vi "HFRR ADV v039.vi"() -> ()   [LabVIEW 2025] (continued)
            n2168 = Bundle "Bundle"(w2334, w2365) -> (w2352:cluster{dbl[], dbl[]})  [unwired: 1 in]
            n2169 = Bundle "Bundle"(w2334, w2419) -> (w2353:cluster{dbl[], dbl[]})  [unwired: 1 in]
            n2170 = Bundle "Bundle"(w2365, w2361) -> (w2367:cluster{dbl[], dbl[]})  [unwired: 1 in]
            n2171 = Bundle "Bundle"(w2330, w2329) -> (w2337:cluster{dbl[], dbl[]})  [unwired: 1 in]
            n2172 = Bundle "Bundle"(w2363, w2359) -> (w2369:cluster{dbl[], dbl[]})  [unwired: 1 in]
            n2173 = Bundle "Bundle"(w2330, w2363) -> (w2473:cluster{dbl[], dbl[]})  [unwired: 1 in]
            n2174 = Bundle "Bundle"(w2330, w2359) -> (w2397:cluster{dbl[], dbl[]})  [unwired: 1 in]
            n2175 = Bundle "Bundle"(w2330, w2418) -> (w2483:cluster{dbl[], dbl[]})  [unwired: 1 in]
            n2176 = Bundle "Bundle"(w2330, w2413) -> (w2421:cluster{dbl[], dbl[]})  [unwired: 1 in]
            n2177 = Bundle "Bundle"(w2330, w2444) -> (w2468:cluster{dbl[], dbl[]})  [unwired: 1 in]
            n2178 = Bundle "Bundle"(w2364, w2360) -> (w2368:cluster{dbl[], dbl[]})  [unwired: 1 in]
            n2179 = Bundle "Bundle"(w2332, w2331) -> (w2338:cluster{dbl[], dbl[]})  [unwired: 1 in]
            n2180 = Bundle "Bundle"(w2332, w2364) -> (w2475:cluster{dbl[], dbl[]})  [unwired: 1 in]
            n2181 = Bundle "Bundle"(w2332, w2360) -> (w2398:cluster{dbl[], dbl[]})  [unwired: 1 in]
            n2182 = Bundle "Bundle"(w2332, w2414) -> (w2422:cluster{dbl[], dbl[]})  [unwired: 1 in]
            n2183 = Bundle "Bundle"(w2332, w2416) -> (w2484:cluster{dbl[], dbl[]})  [unwired: 1 in]
            n2184 = Bundle "Bundle"(w2332, w2453) -> (w2466:cluster{dbl[], dbl[]})  [unwired: 1 in]
            n2185 = Bundle "Bundle"(w2362, w2358) -> (w2370:cluster{dbl[], dbl[]})  [unwired: 1 in]
            n2186 = Bundle "Bundle"(w2328, w2327) -> (w2336:cluster{dbl[], dbl[]})  [unwired: 1 in]
            n2187 = Bundle "Bundle"(w2328, w2362) -> (w2474:cluster{dbl[], dbl[]})  [unwired: 1 in]
            n2188 = Bundle "Bundle"(w2328, w2358) -> (w2396:cluster{dbl[], dbl[]})  [unwired: 1 in]
            n2189 = Bundle "Bundle"(w2328, w2412) -> (w2420:cluster{dbl[], dbl[]})  [unwired: 1 in]
            n2190 = Bundle "Bundle"(w2328, w2417) -> (w2482:cluster{dbl[], dbl[]})  [unwired: 1 in]
            n2191 = Bundle "Bundle"(w2328, w2435) -> (w2467:cluster{dbl[], dbl[]})  [unwired: 1 in]
            n2192 = call-poly <vilib>:"Mean.vi"("X"=w2415) -> ("mean"=→"CP1":dbl)  [unwired: 1 out]
            n2193 = call-poly <vilib>:"Mean.vi"("X"=w2356) -> ("mean"=→"КОФ2 3":dbl)  [unwired: 1 out]
            n2194 = call-poly <vilib>:"Mean.vi"("X"=w2414) -> ("mean"=→"CP2":dbl)  [unwired: 1 out]
            n2195 = call-poly <vilib>:"Mean.vi"("X"=w2416) -> ("mean"=→"КОФ2":dbl)  [unwired: 1 out]
            n2196 = call-poly <vilib>:"Mean.vi"("X"=w2354) -> ("mean"=→"КОФ2 5":dbl)  [unwired: 1 out]
            n2197 = call-poly <vilib>:"Mean.vi"("X"=w2412) -> ("mean"=→"CP4":dbl)  [unwired: 1 out]
            n2198 = call-poly <vilib>:"Mean.vi"("X"=w2417) -> ("mean"=→"КОФ4":dbl)  [unwired: 1 out]
            n2199 = Bundle "Bundle"(w2334, w2361) -> (w2325:cluster{dbl[], dbl[]})  [unwired: 1 in]
            n2200 = Bundle "Bundle"(w2334, w2415) -> (w2348:cluster{dbl[], dbl[]})  [unwired: 1 in]
            n2201 = Build Array "Build Array"(w2325, w2348) -> (w2351:cluster{dbl[], dbl[]}[])
            "XY Graph 17" <- w2351
            n2202 = Build Array "Build Array"(w2339, w2338, w2337, w2336) -> (→"Frequency ( Hz )":cluster{dbl[], dbl[]}[])
            n2203 = Build Array "Build Array"(w2367, w2368, w2369, w2370) -> (→"Air Temp ( °C ) vs Humidity ( % RH )":cluster{dbl[], dbl[]}[])
            n2204 = Build Array "Build Array"(w2352, w2475, w2473, w2474) -> (→"Air Temperature  ( °C )":cluster{dbl[], dbl[]}[])
            n2205 = Build Array "Build Array"(w2325, w2398, w2397, w2396) -> (→"Humidity ( %RH )":cluster{dbl[], dbl[]}[])
            n2206 = Build Array "Build Array"(w2353, w2484, w2483, w2482) -> (→"Coefficient Of Friction":cluster{dbl[], dbl[]}[])
            n2207 = Build Array "Build Array"(w2348, w2422, w2421, w2420) -> (→"Sample Temperature ( °C )":cluster{dbl[], dbl[]}[])
            n2208 = Build Array "Build Array"(w2326, w2466, w2468, w2467) -> (→"XY Graph 13":cluster{dbl[], dbl[]}[])
            n2209 = Bundle "Bundle"(w2334, w2357) -> (w2379:cluster{dbl[], dbl[]})  [unwired: 1 in]
            n2210 = Bundle "Bundle"(w2330, w2355) -> (w2377:cluster{dbl[], dbl[]})  [unwired: 1 in]
            n2211 = Bundle "Bundle"(w2332, w2356) -> (w2378:cluster{dbl[], dbl[]})  [unwired: 1 in]
            n2212 = Bundle "Bundle"(w2328, w2354) -> (w2376:cluster{dbl[], dbl[]})  [unwired: 1 in]
            n2213 = Build Array "Build Array"(w2379, w2378, w2377, w2376) -> (→"Stroke ( mm )":cluster{dbl[], dbl[]}[])
            n2214 = local write "XY Graph 16"(w2351) -> ()
          }
          frame #2 {
          }
          frame #3 {
            n2215 = local write "Numeric 8"(0 ("Numeric 8")) -> ()
            n2216 = local write "Numeric 11"(0 ("Numeric 11")) -> ()
            n2217 = local write "Numeric 12"(0 ("Numeric 12")) -> ()
            n2218 = local write "Numeric 13"(0 ("Numeric 13")) -> ()
            n2219 = property on="OPEN" class="Bool (strict)"("Visible"=TRUE) -> ()  [unwired: 2 in, 2 out]
            n2220 = local read "String Control 2"() -> (w2651:string)
            n2221 = local read "String Control 4"() -> (w2650:string)
            n2222 = local read "String Control 6"() -> (w2649:string)
            n2223 = local read "String Control 8"() -> (w2648:string)
            n2224 = Match Pattern(string=w2651, regular expression="Samples / cycle :- ") -> (after substring=w2665:string)  [unwired: 1 in, 3 out]
            n2225 = Match Pattern(string=w2651, regular expression="Frequency :- ") -> (after substring=w2684:string)  [unwired: 1 in, 3 out]
            n2226 = Match Pattern(string=w2650, regular expression="Samples / cycle :- ") -> (after substring=w2661:string)  [unwired: 1 in, 3 out]
            n2227 = Match Pattern(string=w2650, regular expression="Frequency :- ") -> (after substring=w2679:string)  [unwired: 1 in, 3 out]
            n2228 = Match Pattern(string=w2649, regular expression="Samples / cycle :- ") -> (after substring=w2657:string)  [unwired: 1 in, 3 out]
            n2229 = Match Pattern(string=w2649, regular expression="Frequency :- ") -> (after substring=w2674:string)  [unwired: 1 in, 3 out]
            n2230 = Match Pattern(string=w2648, regular expression="Samples / cycle :- ") -> (after substring=w2653:string)  [unwired: 1 in, 3 out]
            n2231 = Match Pattern(string=w2648, regular expression="Frequency :- ") -> (after substring=w2669:string)  [unwired: 1 in, 3 out]
            n2232 = String Subset(string=w2665, length (rest)=6 ("length (rest)")) -> (substring=w2667:string)  [unwired: 1 in]
            n2233 = String Subset(string=w2684, length (rest)=9 ("length (rest)")) -> (substring=w2686:string)  [unwired: 1 in]
            n2234 = String Subset(string=w2661, length (rest)=6 ("length (rest)")) -> (substring=w2663:string)  [unwired: 1 in]
            n2235 = String Subset(string=w2679, length (rest)=9 ("length (rest)")) -> (substring=w2681:string)  [unwired: 1 in]
            n2236 = String Subset(string=w2657, length (rest)=6 ("length (rest)")) -> (substring=w2659:string)  [unwired: 1 in]
            n2237 = String Subset(string=w2674, length (rest)=9 ("length (rest)")) -> (substring=w2676:string)  [unwired: 1 in]
            n2238 = String Subset(string=w2653, length (rest)=6 ("length (rest)")) -> (substring=w2655:string)  [unwired: 1 in]
            n2239 = String Subset(string=w2669, length (rest)=9 ("length (rest)")) -> (substring=w2671:string)  [unwired: 1 in]
            n2240 = Fract/Exp String To Number(string=w2667) -> (number=w2647:dbl)  [unwired: 3 in, 1 out]
            n2241 = Fract/Exp String To Number(string=w2686) -> (number=w2687:dbl)  [unwired: 3 in, 1 out]
            n2242 = Fract/Exp String To Number(string=w2663) -> (number=w2646:dbl)  [unwired: 3 in, 1 out]
            n2243 = Fract/Exp String To Number(string=w2681) -> (number=w2682:dbl)  [unwired: 3 in, 1 out]
            n2244 = Fract/Exp String To Number(string=w2659) -> (number=w2645:dbl)  [unwired: 3 in, 1 out]
            n2245 = Fract/Exp String To Number(string=w2676) -> (number=w2677:dbl)  [unwired: 3 in, 1 out]
            n2246 = Fract/Exp String To Number(string=w2655) -> (number=w2644:dbl)  [unwired: 3 in, 1 out]
            n2247 = Fract/Exp String To Number(string=w2671) -> (number=w2672:dbl)  [unwired: 3 in, 1 out]
            n2248 = local write "sample1"(w2647) -> ()
            n2249 = local write "freq1"(w2687) -> ()
            n2250 = local write "sample2"(w2646) -> ()
            n2251 = local write "freq2"(w2682) -> ()
            n2252 = local write "sample3"(w2645) -> ()
            n2253 = local write "freq3"(w2677) -> ()
            n2254 = local write "sample4"(w2644) -> ()
            n2255 = local write "freq 4"(w2672) -> ()
          }
        }
      }
    }
    n2256 = case shown="True" w2245 {
      selector: w2245 -> [_ w2264]
      frame False {
      }
      frame True {
        n2257 = Not(x=w2264) -> (.not. x?=w2260:bool)
        n2258 = local write "service 3"(w2260) -> ()
        n2259 = local write "OPEN 6"(w2260) -> ()
        n2260 = call <vilib>:"System Exec.vi"("wait until completion? (T)"=TRUE, "command line"="C:\\LAB-IQ\\Scar View.exe") -> ("error out"=→"error out 5":errorcluster)  [unwired: 6 in, 3 out]
      }
    }
    n2261 = case shown="\"Acquire\", Default" w2254 {
      frame "Acquire", Default {
        # "Elapsed time\ncof\nstroke\nAir temp\nTemp\nHumidity"
        n2262 = disable-structure shown="Disabled" {
          frame Disabled {
            n2263 = local read "Flag"() -> (w2963:dbl)
            n2264 = local read "RUN"() -> (w2960:bool)
            n2265 = Not(x=w2960) -> (.not. x?=w2959:bool)
            n2266 = Equal?(x=w2963, y=10.0) -> (x = y?=w2961:bool)
            n2267 = And(x=w2961, y=w2959) -> (x .and. y?=w2958:bool)
            n2268 = case shown="True" w2958 {
              frame False {
              }
              frame True {
                w2964 = FALSE ("Heater Button")
                n2269 = local write "Humidity"(w2964) -> ()
                n2270 = local write "Heater Button"(w2964) -> ()
              }
            }
          }
          frame Enabled {
          }
        }
        n2271 = disable-structure shown="Disabled" {
          frame Disabled {
            n2272 = case shown="True" {
              selector: _ -> [_ _]
              frame False {
              }
              frame True {
                w3009 = TRUE ("Heater")
                n2273 = local write "Humidity"(w3009) -> ()
                n2274 = local write "Heater Button"(w3009) -> ()
                n2275 = local read "TEST STANDARD"() -> (w3012:T3)
                n2276 = local read "TEST STANDARD"() -> (w3007:T3)
                n2277 = Equal?(x=w3012, y=enum16{"ASTM D6079", "ISO 12156", "Custom"}."ISO 12156" ("Test Standard")) -> (x = y?=w3010:bool)
                n2278 = Equal?(x=w3007, y=enum16{"ASTM D6079", "ISO 12156", "Custom"}."ASTM D6079" ("Test Standard")) -> (x = y?=w3006:bool)
                n2279 = case shown="True" w3010 {
                  frame False {
                  }
                  frame True {
                    n2280 = local write "airtempflg"(FALSE ("airtempflg")) -> ()
                    n2281 = local write item#-1(TRUE ("Heater")) -> ()
                  }
                }
                n2282 = case shown="True" w3006 {
                  frame False {
                  }
                  frame True {
                    n2283 = local write "airtempflg"(TRUE ("airtempflg")) -> ()
                    n2284 = local write item#-1(FALSE ("Heater")) -> ()
                  }
                }
              }
            }
          }
          frame Enabled {
          }
        }
        n2285 = stacked-sequence {
          frame #0 {
            n2286 = case shown="True" "RST FF" {
              frame False {
              }
              frame True {
                w3026 = 0.0 ("X Scale.Range:Maximum")
                n2287 = property on="Frictional Force ( N )" class="WFChart (strict)"("XScale.Maximum"=600.0 ("X Scale.Range:Maximum"), "XScale.Minimum"=w3026, "YScale.Maximum"=10.0 ("Y Scale.Range:Maximum"), "YScale.Minimum"=w3026) -> ()  [unwired: 2 in, 2 out]
              }
            }
          }
          frame #1 {
            n2288 = case shown="True" "RST TEMP" {
              frame False {
              }
              frame True {
                n2289 = property on="Temperature ( Deg C )" class="WFChart (strict)"("XScale.Minimum"=0.0 ("X Scale.Range:Minimum"), "XScale.Maximum"=600.0 ("X Scale.Range:Maximum"), "YScale.Minimum"=0.0 ("Y Scale.Range:Minimum"), "YScale.Maximum"=100.0 ("Y Scale.Range:Maximum")) -> ()  [unwired: 2 in, 2 out]
              }
            }
          }
          frame #2 {
            n2290 = case shown="True" "RSTCOF" {
              frame False {
              }
              frame True {
                n2291 = property on="Coefficient of Friction" class="WFChart (strict)"("XScale.Minimum"=0.0 ("X Scale.Range:Minimum"), "XScale.Maximum"=600.0 ("X Scale.Range:Maximum"), "YScale.Maximum"=1.0 ("X Scale.Range:Minimum"), "YScale.Minimum"=0.0 ("X Scale.Range:Minimum")) -> ()  [unwired: 2 in, 2 out]
              }
            }
          }
          frame #3 {
            n2292 = case shown="True" "RSTCOF 2" {
              frame False {
              }
              frame True {
                (unwired) 100.0 ("Y Scale.Range:Maximum")
                (unwired) 0.0 ("Y Scale.Range:Minimum")
                (unwired) 600.0 ("X Scale.Range:Maximum")
                (unwired) 0.0 ("X Scale.Range:Minimum")
              }
            }
          }
          frame #4 {
            n2293 = case shown="True" "RSTCOF 3" {
              frame False {
              }
              frame True {
                n2294 = property on="Electrical Contact Resistance ( % )" class="WFChart (strict)"("XScale.Minimum"=0.0 ("X Scale.Range:Minimum"), "XScale.Maximum"=600.0 ("X Scale.Range:Maximum"), "YScale.Minimum"=0.0 ("Y Scale.Range:Minimum"), "YScale.Maximum"=100.0 ("Y Scale.Range:Maximum")) -> ()  [unwired: 2 in, 2 out]
              }
            }
          }
        }
        n2295 = local read "RUN"() -> (w2953:bool)
        n2296 = case shown="False" w2953 {
          frame False {
          }
          frame True {
          }
        }
        n2297 = local read "RUN"() -> (w2957:bool)
        n2298 = case shown="False" w2957 {
          tunnel: [FALSE ("TEST RUNNING") TRUE ("TEST RUNNING")] -> w2956
          frame False {
            w3045 = 0.0 ("Flag")
            n2299 = local write "Elapsed time"(0.0 ("elapsedtime")) -> ()
            n2300 = local write "Time Remaining"(w3045) -> ()
            n2301 = local write "Flag"(w3045) -> ()
            n2302 = local write "Remaining Time"(w3045) -> ()
          }
          frame True {
            n2303 = local write "Flag"(10.0 ("Flag")) -> ()
          }
        }
        n2304 = local read "AIR TEMP"() -> (w2951:dbl)
        n2305 = Greater Or Equal?(x=w2951, y=15.0) -> (x >= y?=w2952:bool)
        "powstat" <- w2952
        n2306 = case shown="True" "Save & Continue" {
          frame False {
          }
          frame True {
            n2307 = local read "USER ID"() -> (w3349:string)
            n2308 = local read "FILE"() -> (w3357:string)
            n2309 = String Length(string=w3357) -> (length=w3355:i32)
            n2310 = String Length(string=w3349) -> (length=w3352:i32)
            n2311 = Greater?(x=w3355, y=0) -> (0:w3354:bool)
            n2312 = Greater?(x=w3352, y=0) -> (0:w3351:bool)
            n2313 = And(x=w3354, y=w3351) -> (x .and. y?=w3350:bool)
            n2314 = case shown="True" w3350 {
              frame False {
                n2315 = stacked-sequence {
                  frame #0 {
                    n2316 = One Button Dialog(message="Please Enter a File Name and Operator ID to save data !", button name ("OK")="Ok") -> ()  [unwired: 1 out]
                  }
                  frame #1 {
                    n2317 = local write "Save & Continue"(FALSE ("OK Button")) -> ()
                  }
                }
                n2318 = local write "Save & Continue"(FALSE ("OK Button")) -> ()
              }
              frame True {
                n2319 = stacked-sequence {
                  frame #0 {
                    n2320 = local read "FILE"() -> (w3363:string)
                    n2321 = call "file check.vi"("file name in"=w3363) -> ("file name out"=w3362:string)  [unwired: 9 in, 1 out]
                    n2322 = call <vilib>:"Application Directory.vi"() -> ("Application Directory"=w3373:path)
                    n2323 = Build Path(base path=w3373, name or relative path="data") -> (appended path=w3372:path)
                    n2324 = call <vilib>:"Trim Whitespace.vi"("string"=w3362) -> ("trimmed string"=w3370:string)  [unwired: 1 in]
                    n2325 = call <vilib>:"Trim Whitespace.vi"("string"=w3362) -> ("trimmed string"=w3371:string)  [unwired: 1 in]
                    n2326 = List Folder(path=w3372) -> (folder names=w3368:string[])  [unwired: 3 in, 3 out]
                    n2327 = Match Pattern(string=w3370, regular expression="_(") -> (before substring=w3367:string)  [unwired: 1 in, 3 out]
                    n2328 = for {
                      tunnel: w3368 -> [w3382] mode=indexing
                      tunnel: w3367 -> [w3380]
                      shift-right: [w3378] -> w3365
                      shift-left: bool[] [] -> [w3379]
                      n2329 = Match Pattern(string=w3382, regular expression="_(") -> (before substring=w3381:string)  [unwired: 1 in, 3 out]
                      n2330 = Equal?(x=w3381, y=w3380) -> (x = y?=w3377:bool)
                      n2331 = case shown="True" w3377 {
                        tunnel: w3377 -> [_ w3385]
                        tunnel: w3379 -> [w3384 w3387]
                        tunnel: [w3384 w3386] -> w3378
                        frame False {
                        }
                        frame True {
                          n2332 = Insert Into Array(array=w3387, new element=w3385) -> (w3386:bool[])  [unwired: 1 in]
                        }
                      }
                    }
                    n2333 = Equal?(x=w3368, y=w3367) -> (x = y?=w3376:bool[])
                    n2334 = Or Array Elements(Boolean array=w3376) -> (logical OR=w3375:bool)
                    n2335 = Array Size(array=w3365) -> (size(s)=w3364:i32)
                    n2336 = case shown="True" w3375 {
                      tunnel: w3371 -> [_ w3395]
                      tunnel: w3364 -> [_ w3388]
                      frame False {
                      }
                      frame True {
                        n2337 = Number To Decimal String(number=w3388) -> (decimal integer string=w3391:string)  [unwired: 1 in]
                        n2338 = Search/Split String(string=w3395, search string/char (-)="_(" ("regular expression")) -> (substring before match=w3393:string)  [unwired: 1 in, 2 out]
                        n2339 = Concatenate Strings(w3393, "_(" ("regular expression"), w3391, ")" ("regular expression")) -> (w3389:string)
                        n2340 = local write "FILE"(w3389) -> ()
                      }
                    }
                  }
                  frame #1 {
                    w3398 = 0.0
                    w3411 = cluster{"y":dbl, dbl, "y":dbl}[] [] ("History Data")
                    w3412 = FALSE ("Heater Button")
                    (unwired) ")!" ("string")
                    (unwired) ")" ("string")
                    w3410 = dbl[] [] ("History Data")
                    w3416 = "\r"
                    # "C:\\WinDucom\\Data\\"
                    # "C:\\LAB-IQ-NXT\\data"
                    n2341 = local write "Humidity ( %RH )"(w3398) -> ()
                    n2342 = local write "Frequency ( Hz )"(w3398) -> ()
                    n2343 = local write "Stroke 3"(w3398) -> ()
                    n2344 = local write "speedop"(0.0 ("PIDclk 2")) -> ()
                    n2345 = local write "Set Temp 2"(65.0 ("Set Temp 2")) -> ()
                    n2346 = local write "AIR TEMP"(w3398) -> ()
                    n2347 = local write "clk"(0.0 ("clk")) -> ()
                    n2348 = local write "Stroke 4"(w3398) -> ()
                    n2349 = local write "COF 2"(w3398) -> ()
                    n2350 = local write "TEMP"(w3398) -> ()
                    n2351 = local write "ecr 3"(w3398) -> ()
                    n2352 = local write "FF 3"(w3398) -> ()
                    n2353 = local write "FF 2"(w3398) -> ()
                    n2354 = property on="Coefficient of Friction" class="WFChart (strict)"("History Data"=w3410) -> ()  [unwired: 2 in, 2 out]
                    n2355 = property on="Coefficient of Friction" class="WFChart (strict)"("History Data"=w3410) -> ()  [unwired: 2 in, 2 out]
                    n2356 = property on="Frictional Force ( N )" class="WFChart (strict)"("History Data"=w3410) -> ()  [unwired: 2 in, 2 out]
                    n2357 = property on="Electrical Contact Resistance ( % )" class="WFChart (strict)"("History Data"=w3410) -> ()  [unwired: 2 in, 2 out]
                    n2358 = property on="Electrical Contact Resistance ( % )" class="WFChart (strict)"("History Data"=w3410) -> ()  [unwired: 2 in, 2 out]
                    n2359 = property on="Temperature ( Deg C )" class="WFChart (strict)"("History Data"=w3410) -> ()  [unwired: 2 in, 2 out]
                    n2360 = property on="Frictional Force ( N )" class="WFChart (strict)"("History Data"=w3410) -> ()  [unwired: 2 in, 2 out]
                    n2361 = property on="Coefficient of Friction" class="WFChart (strict)"("History Data"=w3410) -> ()  [unwired: 2 in, 2 out]
                    n2362 = property on="Frictional Force ( N )" class="WFChart (strict)"("History Data"=w3410) -> ()  [unwired: 2 in, 2 out]
                    n2363 = property on="Electrical Contact Resistance ( % )" class="WFChart (strict)"("History Data"=w3410) -> ()  [unwired: 2 in, 2 out]
                    n2364 = property on="Temperature ( Deg C )" class="WFChart (strict)"("History Data"=w3410) -> ()  [unwired: 2 in, 2 out]
                    n2365 = property on="Stroke ( mm )" class="WFChart (strict)"("History Data"=w3411) -> ()  [unwired: 2 in, 2 out]
                    n2366 = property on="Stroke ( mm )" class="WFChart (strict)"("History Data"=w3411) -> ()  [unwired: 2 in, 2 out]
                    n2367 = local write "Humidity"(w3412) -> ()
                    n2368 = local write "Heater Button"(w3412) -> ()
                    n2369 = local read "FILE"() -> (w3406:string)
                    n2370 = disable-structure shown="Enabled" {
                      disable-tunnel: [w3450 _] -> w3397
                      frame Enabled {
                        n2371 = local read "NORMAL LOAD"() -> (w3450:dbl)
                      }
                      frame Disabled {
                      }
                    }
                    n2372 = call "file check.vi"("file name in"=w3406) -> ("error out"=w3409:errorcluster, "file name out"=w3403:string)  [unwired: 9 in]
                    n2373 = call "FILE PATH CREATION.vi"("error in"=w3409, "FILE NAME :"=w3403) -> ("FILE OUT"=w3402:path)  [unwired: 8 in, 1 out]
                    n2374 = Concatenate Strings(w3403, ".dgf" ("Substring")) -> (w3408:string)
                    n2375 = Concatenate Strings(w3403, ".duf" ("Substring")) -> (w3404:string)
                    n2376 = Multiply(x=w3397, y=1.0) -> (x*y=w3429:dbl)
                    n2377 = Build Path(base path=w3402, name or relative path=w3408) -> (appended path=w3401:path)
                    n2378 = Build Path(base path=w3402, name or relative path=w3404) -> (appended path=w3400:path)
                    n2379 = Number To Fractional String(number=w3429, width (-)=i16 5, precision (6)=i16 2) -> (F-format string=w3437:string)  [unwired: 1 in]
                    n2380 = local read "tested by"() -> (w3396:string)
                    n2381 = local read "Fuel Discription :"() -> (w3425:string)
                    n2382 = local read "Batch Ref Num :"() -> (w3414:string)
                    n2383 = Get Date/Time String(date format (0)=enum16{"short", "long", "abbreviated"}."short") -> (date string=w3448:string, time string=w3445:string)  [unwired: 2 in]
                    n2384 = local read "Remarks :"() -> (w3424:string)
                    n2385 = Concatenate Strings("Load :- " ("Substring"), w3437, " grams ," ("Substring")) -> (w3436:string)
                    n2386 = local read "String 41"() -> (w3417:string)
                    n2387 = Concatenate Strings(w3425) -> (w3426:string)
                    n2388 = Concatenate Strings(w3414) -> (w3413:string)
                    n2389 = Concatenate Strings(w3396) -> (w3420:string)
                    n2390 = Concatenate Strings("(" ("Substring"), w3448, ")" ("Substring"), w3445) -> (w3419:string)
                    "concatenated string" <- w3419
                    n2391 = Concatenate Strings(w3424, "," ("string")) -> (w3423:string)
                    n2392 = Concatenate Strings("  TIME;      COF;       STROKE;     AIR TEMP;  TEMP;  HUMIDITY;  ECR; PID-OUT; FREQUENCY" ("Substring"), "\r") -> (w3432:string)
                    n2393 = Concatenate Strings(w3417, w3416, "Fuel Discription :-" ("Substring"), w3426, w3416, w3436, w3416, "Batch Ref Num :-" ("Substring"), w3413, w3416, " Remarks :- " ("Substring"), w3423, w3416, " Date :- " ("Substring"), w3419, w3416, "Tested By :-" ("Substring"), w3420) -> (w3430:string)
                    "REMARKS" <- w3430
                    n2394 = call <vilib>:"Write Characters To File.vi"("append to file? (new file:F)"=FALSE, "character string"=w3432, "file path (dialog if empty)"=w3401) -> ()  [unwired: 2 in, 1 out]
                    n2395 = call <vilib>:"Write Characters To File.vi"("append to file? (new file:F)"=FALSE, "character string"=w3430, "file path (dialog if empty)"=w3400) -> ()  [unwired: 2 in, 1 out]
                  }
                  frame #2 {
                    n2396 = local write "Cycles elapsed"(0 ("Cycles elapsed")) -> ()
                    n2397 = local write "cyclecount"(0 ("cyclecount")) -> ()
                    n2398 = local write "Save & Continue"(FALSE ("OK")) -> ()
                    n2399 = local write "autostrtflg"(TRUE ("autostrtflg")) -> ()
                    n2400 = local write "Save"(FALSE ("Save")) -> ()
                    n2401 = Get Date/Time In Seconds() -> (seconds since 1Jan1904=w3455:timestamp)
                    n2402 = To Double Precision Float(number=w3455) -> (double precision float=w3454:dbl)
                    n2403 = local write "acq timer"(w3454) -> ()
                    n2404 = One Button Dialog(message="Please ensure sample is mounted properly and machine is ready in all aspects for testing !", button name ("OK")="Ok") -> ()  [unwired: 1 out]
                  }
                  frame #3 {
                    n2405 = stacked-sequence {
                      frame #0 {
                        n2406 = local write "Main Dashboard Buttons"(T1."Dashboard" ("Main Dashboard Buttons")) -> ()
                        n2407 = local write "Main Tab"(T2."Acquire" ("Main Tab")) -> ()
                      }
                      frame #1 {
                        n2408 = local write "EVENT LOG"("" ("EVENT LOG")) -> ()
                      }
                      frame #2 {
                        n2409 = Wait (ms)(milliseconds to wait=u32 50) -> ()  [unwired: 1 out]
                      }
                      frame #3 {
                        n2410 = disable-structure shown="Disabled" {
                          frame Disabled {
                            n2411 = local read "EVENT LOG"() -> (w3467:string)
                            n2412 = call "Event Log.vi"("Content"="Test Details", "EVENT LOG"=w3467) -> ("EVENT LOG"=w3466:string)  [unwired: 8 in, 1 out]
                            n2413 = local write "EVENT LOG"(w3466) -> ()
                          }
                          frame Enabled {
                          }
                        }
                      }
                      frame #4 {
                        n2414 = Wait (ms)(milliseconds to wait=u32 50) -> ()  [unwired: 1 out]
                      }
                      frame #5 {
                        n2415 = local read "FILE"() -> (w3469:string)
                        n2416 = Concatenate Strings("File Name :" ("Content"), w3469) -> (w3470:string)
                        n2417 = local read "EVENT LOG"() -> (w3473:string)
                        n2418 = call "Event Log.vi"("Content"=w3470, "EVENT LOG"=w3473) -> ("EVENT LOG"=w3472:string)  [unwired: 8 in, 1 out]
                        n2419 = local write "EVENT LOG"(w3472) -> ()
                      }
                      frame #6 {
                        n2420 = Wait (ms)(milliseconds to wait=u32 50) -> ()  [unwired: 1 out]
                      }
                      frame #7 {
                        n2421 = local read "Batch Ref Num :"() -> (w3475:string)
                        n2422 = Concatenate Strings("Batch Ref No :" ("Content"), w3475) -> (w3476:string)
                        n2423 = local read "EVENT LOG"() -> (w3479:string)
                        n2424 = call "Event Log.vi"("Content"=w3476, "EVENT LOG"=w3479) -> ("EVENT LOG"=w3478:string)  [unwired: 8 in, 1 out]
                        n2425 = local write "EVENT LOG"(w3478) -> ()
                      }
                      frame #8 {
                        n2426 = Wait (ms)(milliseconds to wait=u32 50) -> ()  [unwired: 1 out]
                      }
                      frame #9 {
                        n2427 = local read "tested by"() -> (w3481:string)
                        n2428 = Concatenate Strings("Tested By :" ("Content"), w3481) -> (w3482:string)
                        n2429 = local read "EVENT LOG"() -> (w3485:string)
                        n2430 = call "Event Log.vi"("Content"=w3482, "EVENT LOG"=w3485) -> ("EVENT LOG"=w3484:string)  [unwired: 8 in, 1 out]
                        n2431 = local write "EVENT LOG"(w3484) -> ()
                      }
                      frame #10 {
                        n2432 = Wait (ms)(milliseconds to wait=u32 50) -> ()  [unwired: 1 out]
                      }
                      frame #11 {
                        n2433 = local read "TEST STANDARD"() -> (w3488:T3)
                        n2434 = case shown="\"ASTM D6079\", Default" w3488 {
                          tunnel: ["ASTM D6079" "ISO 12156" "CEC F-096-A-06" "Custom"] -> w3487
                          frame "ASTM D6079", Default {
                          }
                          frame "ISO 12156" {
                          }
                          frame "CEC F-096-A-06" {
                          }
                          frame "Custom" {
                          }
                        }
                        n2435 = Concatenate Strings("Test Standard :" ("Content"), w3487) -> (w3489:string)
                        n2436 = local read "EVENT LOG"() -> (w3492:string)
                        n2437 = call "Event Log.vi"("Content"=w3489, "EVENT LOG"=w3492) -> ("EVENT LOG"=w3491:string)  [unwired: 8 in, 1 out]
                        n2438 = local write "EVENT LOG"(w3491) -> ()
                      }
                      frame #12 {
                        n2439 = Wait (ms)(milliseconds to wait=u32 50) -> ()  [unwired: 1 out]
                      }
                      frame #13 {
                        n2440 = local read "Fuel Discription :"() -> (w3498:string)
                        n2441 = Concatenate Strings("Fuel Description :" ("Content"), w3498) -> (w3499:string)
                        n2442 = local read "EVENT LOG"() -> (w3502:string)
                        n2443 = call "Event Log.vi"("Content"=w3499, "EVENT LOG"=w3502) -> ("EVENT LOG"=w3501:string)  [unwired: 8 in, 1 out]
                        n2444 = local write "EVENT LOG"(w3501) -> ()
                      }
                      frame #14 {
                        n2445 = Wait (ms)(milliseconds to wait=u32 50) -> ()  [unwired: 1 out]
                      }
                      frame #15 {
                        n2446 = local read "Remarks :"() -> (w3504:string)
                        n2447 = Concatenate Strings("Remarks :" ("Content"), w3504) -> (w3505:string)
                        n2448 = local read "EVENT LOG"() -> (w3508:string)
                        n2449 = call "Event Log.vi"("Content"=w3505, "EVENT LOG"=w3508) -> ("EVENT LOG"=w3507:string)  [unwired: 8 in, 1 out]
                        n2450 = local write "EVENT LOG"(w3507) -> ()
                      }
                      frame #16 {
                        n2451 = Wait (ms)(milliseconds to wait=u32 50) -> ()  [unwired: 1 out]
                      }
                      frame #17 {
                        n2452 = local read "USER ID"() -> (w3510:string)
                        n2453 = Concatenate Strings("Operator ID :" ("Content"), w3510) -> (w3512:string)
                        n2454 = local read "EVENT LOG"() -> (w3514:string)
                        n2455 = call "Event Log.vi"("Content"=w3512, "EVENT LOG"=w3514) -> ("EVENT LOG"=w3513:string)  [unwired: 8 in, 1 out]
                        n2456 = local write "EVENT LOG"(w3513) -> ()
                      }
                      frame #18 {
                        n2457 = Wait (ms)(milliseconds to wait=u32 50) -> ()  [unwired: 1 out]
                      }
                      frame #19 {
                        n2458 = disable-structure shown="Disabled" {
                          frame Disabled {
                            n2459 = local read "EVENT LOG"() -> (w3518:string)
                            n2460 = call "Event Log.vi"("Content"="Test Parameter", "EVENT LOG"=w3518) -> ("EVENT LOG"=w3517:string)  [unwired: 8 in, 1 out]
                            n2461 = local write "EVENT LOG"(w3517) -> ()
                          }
                          frame Enabled {
                          }
                        }
                      }
                      frame #20 {
                        n2462 = Wait (ms)(milliseconds to wait=u32 50) -> ()  [unwired: 1 out]
                      }
                      frame #21 {
                        n2463 = local read "Set Hz"() -> (w3522:dbl)
                        n2464 = Number To Fractional String(number=w3522, precision (6)=i16 2) -> (F-format string=w3521:string)  [unwired: 2 in]
                        n2465 = Concatenate Strings("Set Frequency [Hz] :" ("Content"), w3521) -> (w3524:string)
                        n2466 = local read "EVENT LOG"() -> (w3526:string)
                        n2467 = call "Event Log.vi"("Content"=w3524, "EVENT LOG"=w3526) -> ("EVENT LOG"=w3525:string)  [unwired: 8 in, 1 out]
                        n2468 = local write "EVENT LOG"(w3525) -> ()
                      }
                      frame #22 {
                        n2469 = Wait (ms)(milliseconds to wait=u32 50) -> ()  [unwired: 1 out]
                      }
                      frame #23 {
                        n2470 = local read "NORMAL LOAD"() -> (w3529:dbl)
                        n2471 = Number To Fractional String(number=w3529, precision (6)=i16 2) -> (F-format string=w3530:string)  [unwired: 2 in]
                        n2472 = Concatenate Strings("Applied Load [grams] :" ("Content"), w3530) -> (w3532:string)
                        n2473 = local read "EVENT LOG"() -> (w3534:string)
                        n2474 = call "Event Log.vi"("Content"=w3532, "EVENT LOG"=w3534) -> ("EVENT LOG"=w3533:string)  [unwired: 8 in, 1 out]
                        n2475 = local write "EVENT LOG"(w3533) -> ()
                      }
                      frame #24 {
                        n2476 = Wait (ms)(milliseconds to wait=u32 50) -> ()  [unwired: 1 out]
                      }
                      frame #25 {
                        n2477 = local read "Set Strk"() -> (w3537:dbl)
                        n2478 = Number To Fractional String(number=w3537, precision (6)=i16 2) -> (F-format string=w3538:string)  [unwired: 2 in]
                        n2479 = Concatenate Strings("Set Stroke [mm] :" ("Content"), w3538) -> (w3540:string)
                        n2480 = local read "EVENT LOG"() -> (w3542:string)
                        n2481 = call "Event Log.vi"("Content"=w3540, "EVENT LOG"=w3542) -> ("EVENT LOG"=w3541:string)  [unwired: 8 in, 1 out]
                        n2482 = local write "EVENT LOG"(w3541) -> ()
                      }
                      frame #26 {
                        n2483 = Wait (ms)(milliseconds to wait=u32 50) -> ()  [unwired: 1 out]
                      }
                      frame #27 {
                        n2484 = local read "Set Temp"() -> (w3545:dbl)
                        n2485 = Number To Fractional String(number=w3545, precision (6)=i16 2) -> (F-format string=w3546:string)  [unwired: 2 in]
                        n2486 = Concatenate Strings("Set Temperature [deg C] :" ("Content"), w3546) -> (w3548:string)
                        n2487 = local read "EVENT LOG"() -> (w3550:string)
                        n2488 = call "Event Log.vi"("Content"=w3548, "EVENT LOG"=w3550) -> ("EVENT LOG"=w3549:string)  [unwired: 8 in, 1 out]
                        n2489 = local write "EVENT LOG"(w3549) -> ()
                      }
                      frame #28 {
                        n2490 = Wait (ms)(milliseconds to wait=u32 50) -> ()  [unwired: 1 out]
                      }
                      frame #29 {
                        n2491 = local read "Set Rh"() -> (w3553:dbl)
                        n2492 = Number To Fractional String(number=w3553, precision (6)=i16 2) -> (F-format string=w3554:string)  [unwired: 2 in]
                        n2493 = Concatenate Strings("Set Humidity [%RH] :" ("Content"), w3554) -> (w3556:string)
                        n2494 = local read "EVENT LOG"() -> (w3558:string)
                        n2495 = call "Event Log.vi"("Content"=w3556, "EVENT LOG"=w3558) -> ("EVENT LOG"=w3557:string)  [unwired: 8 in, 1 out]
                        n2496 = local write "EVENT LOG"(w3557) -> ()
                      }
                      frame #30 {
                        n2497 = Wait (ms)(milliseconds to wait=u32 50) -> ()  [unwired: 1 out]
                      }
                      frame #31 {
                        n2498 = local read "test time"() -> (w3561:dbl)
                        n2499 = Number To Fractional String(number=w3561, precision (6)=i16 1) -> (F-format string=w3562:string)  [unwired: 2 in]
                        n2500 = Concatenate Strings("Test Duration [mins] :" ("Content"), w3562) -> (w3564:string)
                        n2501 = local read "EVENT LOG"() -> (w3566:string)
                        n2502 = call "Event Log.vi"("Content"=w3564, "EVENT LOG"=w3566) -> ("EVENT LOG"=w3565:string)  [unwired: 8 in, 1 out]
                        n2503 = local write "EVENT LOG"(w3565) -> ()
                      }
                      frame #32 {
                        w3567 = dbl[] [] ("History Data")
                        w3568 = cluster{"y":dbl, dbl, "y":dbl}[] [] ("History Data")
                        w3569 = FALSE ("Visible")
                        n2504 = property on="Stroke ( mm )" class="WFChart (strict)"("History Data"=w3568) -> ()  [unwired: 2 in, 2 out]
                        n2505 = property on="Temperature ( Deg C )" class="WFChart (strict)"("History Data"=w3567) -> ()  [unwired: 2 in, 2 out]
                        n2506 = property on="Electrical Contact Resistance ( % )" class="WFChart (strict)"("History Data"=w3567) -> ()  [unwired: 2 in, 2 out]
                        n2507 = property on="Coefficient of Friction" class="WFChart (strict)"("History Data"=w3567) -> ()  [unwired: 2 in, 2 out]
                        n2508 = property on="Frictional Force ( N )" class="WFChart (strict)"("History Data"=w3567) -> ()  [unwired: 2 in, 2 out]
                        n2509 = property on="Coefficient of Friction" class="WFChart (strict)"("History Data"=w3567) -> ()  [unwired: 2 in, 2 out]
                        n2510 = property on="Frictional Force ( N )" class="WFChart (strict)"("History Data"=w3567) -> ()  [unwired: 2 in, 2 out]
                        n2511 = property on="Electrical Contact Resistance ( % )" class="WFChart (strict)"("History Data"=w3567) -> ()  [unwired: 2 in, 2 out]
                        n2512 = property on="Stroke ( mm )" class="WFChart (strict)"("History Data"=w3568) -> ()  [unwired: 2 in, 2 out]
                        n2513 = property on="Temperature ( Deg C )" class="WFChart (strict)"("History Data"=w3567) -> ()  [unwired: 2 in, 2 out]
                        n2514 = property on="Service Password Log" class="Str"("Visible"=w3569) -> ()  [unwired: 2 in, 2 out]
                        n2515 = property on="Password 3" class="Clust (strict)"("Visible"=w3569) -> ()  [unwired: 2 in, 2 out]
                      }
                    }
                    "TEST FILE NAM,E SAVED" <- TRUE ("TEST FILE NAM,E SAVED")
                  }
                }
              }
            }
          }
        }
        n2516 = local write "Test \nStatus"(w2956) -> ()
        n2517 = local write "Save"(w2956) -> ()
        n2518 = local read "Main Tab"() -> (w2950:T2)
        n2519 = case shown="True" w2953 {
          frame False {
            n2520 = local read "Rt 3"() -> (w3017:bool)
            n2521 = case shown="True" w3017 {
              frame False {
              }
              frame True {
                n2522 = local write "Rt 3"(FALSE ("Rt 3")) -> ()
              }
            }
            "Rt" <- TRUE ("Rt")
            "Rt 2" <- FALSE ("Rt")
          }
          frame True {
            n2523 = local read "Rt"() -> (w3023:bool)
            n2524 = local write "Rt 2"(TRUE ("Rt 2")) -> ()
            n2525 = case shown="True" w3023 {
              frame False {
              }
              frame True {
                n2526 = local write "Rt"(FALSE ("Rt")) -> ()
              }
            }
            "Rt 3" <- TRUE ("Rt 3")
          }
        }
        n2527 = case shown="\"Acquire\"" w2950 {
          tunnel: w2952 -> [_ w3052]
          frame Default {
            w3051 = 0.0 ("output")
            n2528 = local write "PID-out"(w3051) -> ()
            n2529 = local write "Frequency ( Hz )"(w3051) -> ()
            n2530 = local write "STROKE Initialize"(TRUE ("STROKE Initialize")) -> ()
          }
          frame "Acquire" {
            n2531 = stacked-sequence {
              frame #0 {
                n2532 = local read "Auto Start Test"() -> (w3054:bool)
                n2533 = case shown="True" w3054 {
                  tunnel: "RUN" -> [w3075 w3078]
                  tunnel: [w3075 w3077] -> w3055
                  frame False {
                  }
                  frame True {
                    n2534 = local read "Auto Start Temp"() -> (w3076:bool)
                    n2535 = Or(x=w3078, y=w3076) -> (x .or. y?=w3077:bool)
                  }
                }
                n2536 = local read "clk"() -> (w3074:dbl)
                n2537 = local read "Save"() -> (w3070:bool)
                n2538 = Equal?(x=w3074, y=0.0) -> (x = y?=w3071:bool)
                n2539 = And(x=w3071, y=w3070) -> (x .and. y?=w3072:bool)
                n2540 = Not(x="Engage") -> (.not. x?=w3061:bool)
                n2541 = case shown="False" w3055 {
                  tunnel: [0.0 w3102] -> w3057
                  frame False {
                    (unwired) TRUE ("Visible")
                    n2542 = local read "Auto Start Test"() -> (w3082:bool)
                    n2543 = local write "Start Time"(TRUE ("Start Time")) -> ()
                    n2544 = property on="Stroke 2" class="DigNum (strict)"("Visible"=FALSE) -> ()  [unwired: 2 in, 2 out]
                    n2545 = case shown="False" w3082 {
                      frame False {
                        n2546 = property on="Heater Button" class="Bool (strict)"("DisabledEnum"=T19."Enabled" ("Disabled")) -> ()  [unwired: 2 in, 2 out]
                        n2547 = property on="Humidity" class="Bool (strict)"("DisabledEnum"=T19."Enabled" ("Disabled")) -> ()  [unwired: 2 in, 2 out]
                      }
                      frame True {
                      }
                    }
                    n2548 = case shown="False" "TestCompFlg" {
                      frame False {
                        n2549 = local read "StartFlg"() -> (w3090:bool)
                        n2550 = case shown="True" w3090 {
                          frame False {
                          }
                          frame True {
                            n2551 = stacked-sequence {
                              frame #0 {
                                n2552 = local read "EVENT LOG"() -> (w3094:string)
                                n2553 = call "Event Log.vi"("Content"="Test was interrupted", "EVENT LOG"=w3094) -> ("EVENT LOG"=w3095:string)  [unwired: 8 in, 1 out]
                                n2554 = local write "EVENT LOG"(w3095) -> ()
                                n2555 = property on="RUN" class="Bool (strict)"("Visible"=TRUE) -> ()  [unwired: 2 in, 2 out]
                                n2556 = property on="Auto Start Test" class="Bool (strict)"("Visible"=TRUE) -> ()  [unwired: 2 in, 2 out]
                              }
                              frame #1 {
                                w3098 = FALSE ("StartFlg")
                                n2557 = property on="Heater Button" class="Bool (strict)"("Val(Sgnl)"=FALSE ("Value (Signaling)")) -> ()  [unwired: 2 in, 2 out]
                                n2558 = local write "Heater Button"(w3098) -> ()
                                n2559 = local write "StartFlg"(w3098) -> ()
                                n2560 = local write "Humidity"(w3098) -> ()
                                n2561 = local write "Humidity 2"(TRUE ("Humidity")) -> ()
                              }
                              frame #2 {
                                n2562 = local write "Due Write"("VC;0" ("Command")) -> ()
                              }
                              frame #3 {
                                n2563 = Wait (ms)(milliseconds to wait=u32 1500) -> ()  [unwired: 1 out]
                              }
                              frame #4 {
                                n2564 = local write "Due Write"("HE;0" ("Command")) -> ()
                              }
                            }
                          }
                        }
                      }
                      frame True {
                      }
                    }
                    n2565 = local write "String 14"("Test will autostart once parameters reach the set value." ("String 14")) -> ()
                  }
                  frame True {
                    (unwired) FALSE ("Visible")
                    n2566 = property on="Stroke 2" class="DigNum (strict)"("Visible"=TRUE) -> ()  [unwired: 2 in, 2 out]
                    n2567 = property on="STOP 2" class="Bool (strict)"("Disabled"=u8 2) -> ()  [unwired: 2 in, 2 out]
                    n2568 = local write "String 14"(" Running....." ("String 14")) -> ()
                    n2569 = property on="Heater Button" class="Bool (strict)"("DisabledEnum"=T19."Disabled and Grayed Out" ("Disabled")) -> ()  [unwired: 2 in, 2 out]
                    n2570 = property on="Humidity" class="Bool (strict)"("DisabledEnum"=T19."Disabled and Grayed Out" ("Disabled")) -> ()  [unwired: 2 in, 2 out]
                    n2571 = case shown="True" "Start Time" {
                      selector: "Start Time" -> [_ w3121]
                      frame False {
                      }
                      frame True {
                        n2572 = Not(x=w3121) -> (.not. x?=w3120:bool)
                        n2573 = local write "Start Time"(w3120) -> ()
                        n2574 = local read "EVENT LOG"() -> (w3122:string)
                        n2575 = call "Event Log.vi"("Content"="Test in progress", "EVENT LOG"=w3122) -> ("EVENT LOG"=w3124:string)  [unwired: 8 in, 1 out]
                        n2576 = local write "EVENT LOG"(w3124) -> ()
                      }
                    }
                    n2577 = disable-structure shown="Enabled" {
                      disable-tunnel: [w3113 w3119] -> w3102
                      frame Disabled {
                        n2578 = local read "Set Hz"() -> (w3116:dbl)
                        n2579 = call <vilib>:"Uniform White Noise Waveform.vi"() -> ("signal out"=w3115:waveform(dbl))  [unwired: 10 in, 1 out]
                        n2580 = Random Number (0-1)() -> (number: 0 to 1=w3112:dbl)
                        n2581 = Add(x=w3116, y=w3115) -> (x+y=w3114:waveform(dbl))
                        n2582 = Multiply(x=ext 0.01 ("y"), y=w3112) -> (x*y=w3110:ext)
                        n2583 = Multiply(x=w3114, y=w3110) -> (x*y=w3113:waveform(ext))
                      }
                      frame Enabled {
                        n2584 = call-poly <vilib>:"Random Number (Range).vi"("lower bound (0)"=49.89, "upper bound (100)"=50.8) -> ("number"=w3119:dbl)  [unwired: 9 in]
                      }
                    }
                    "StartFlg" <- TRUE ("StartFlg")
                  }
                }
                n2585 = case shown="True" w3072 {
                  frame False {
                  }
                  frame True {
                    n2586 = local write "clk"(10.0 ("clk")) -> ()
                    n2587 = Get Date/Time In Seconds() -> (seconds since 1Jan1904=w3127:timestamp)
                    n2588 = To Double Precision Float(number=w3127) -> (double precision float=w3125:dbl)
                    n2589 = local write "acq timer"(w3125) -> ()
                    n2590 = local write "act save time"(w3125) -> ()
                  }
                }
                n2591 = call "Elapsed Time"("Time Target (s)"="Countdown", "Reset"=w3061) -> ("Elapsed Time (s)"=w3066:dbl, "Time has Elapsed"=w3064:bool)  [unwired: 10 in, 6 out]
                "Countdown 2" <- w3066
                n2592 = Subtract(x=w3066, y=2.0) -> (x-y=w3069:dbl)
                n2593 = Less?(x=w3069, y="Countdown") -> (x < y?=w3067:bool)
                n2594 = And(x=w3067, y=w3064) -> (x .and. y?=w3063:bool)
                n2595 = case shown="True" w3063 {
                  frame False {
                  }
                  frame True {
                    (unwired) dbl[] [] ("History Data")
                    n2596 = local write "Engage"(FALSE ("Engage")) -> ()
                    n2597 = local write "RUN"(TRUE ("RUN")) -> ()
                    n2598 = local read "Humidity ( %RH )"() -> (→"Rh Before":dbl)
                  }
                }
                n2599 = local read "Test \nStatus"() -> (w3059:bool)
                n2600 = Select(t=w3057, s=w3059, f=0.0) -> (s? t:f=w3058:dbl)
                n2601 = local write "Frequency ( Hz )"(w3058) -> ()
              }
              frame #1 {
                w3150 = 1000000.0 ("x")
                # "HC;1/0\nST;VALUE"
                # "Elapsed time\ncof\nstroke\nAir temp\nTemp\nHumidity"
                # "acq timer\n\nact save time"
                # "convert to microseconds"
                n2602 = local read "COUNT"() -> (w3133:i32)
                n2603 = local read "Rate"() -> (w3146:dbl)
                n2604 = Divide(x=w3150, y=w3146) -> (x/y=w3151:dbl)
                n2605 = Greater Or Equal?(x=w3133, y=250) -> (x >= y?=w3132:bool)
                n2606 = Get Date/Time In Seconds() -> (seconds since 1Jan1904=w3153:timestamp)
                n2607 = case shown="True" w3132 {
                  frame False {
                    n2608 = local read "COUNT"() -> (w3154:i32)
                    n2609 = Increment(x=w3154) -> (x+1=w3155:i32)
                    n2610 = local write "COUNT"(w3155) -> ()
                  }
                  frame True {
                    n2611 = local write "COUNT"(0 ("COUNT")) -> ()
                  }
                }
                n2612 = local read "Samplingtime 2"() -> (w3131:dbl)
                n2613 = local read "act save time"() -> (w3148:dbl)
                n2614 = Divide(x=w3151, y=w3150) -> (x/y=w3149:dbl)
                n2615 = To Double Precision Float(number=w3153) -> (double precision float=w3142:dbl)
                n2616 = Add(x=w3148, y=w3131) -> (x+y=w3147:dbl)
                n2617 = local read "acq timer"() -> (w3152:dbl)
                n2618 = local read "COUNT"() -> (w3135:i32)
                n2619 = Greater Or Equal?(x=w3142, y=w3147) -> (x >= y?=w3130:bool)
                n2620 = Multiply(x=w3149, y=w3135) -> (x*y=w3141:dbl)
                n2621 = Subtract(x=w3142, y=w3152) -> (x-y=w3144:dbl)
                n2622 = local read "Save"() -> (w3145:bool)
                n2623 = Add(x=w3144, y=w3141) -> (x+y=w3128:dbl)
                "Elapsed time 3" <- w3128
                n2624 = And(x=w3130, y=w3145) -> (x .and. y?=w3143:bool)
                n2625 = Divide(x=w3128, y=60.0) -> (x/y=w3139:dbl)
                n2626 = local read "Test \nStatus"() -> (w3129:bool)
                n2627 = local read "clk"() -> (w3136:dbl)
                n2628 = Equal?(x=w3136, y=10.0) -> (x = y?=w3138:bool)
                n2629 = case shown="True" w3143 {
                  tunnel: w3142 -> [_ w3269]
                  tunnel: [FALSE ("Boolean 2") TRUE ("Boolean 2")] -> _
                  frame False {
                  }
                  frame True {
                    w3223 = ";" ("Substring")
                    # "Pid out/\nFreq response value"
                    n2630 = local write "act save time"(w3269) -> ()
                    n2631 = local read "FILE"() -> (w3217:string)
                    n2632 = call "file check.vi"("file name in"=w3217) -> ("error out"=w3220:errorcluster, "file name out"=w3215:string)  [unwired: 9 in]
                    n2633 = local read "LVDT STROKE"() -> (w3212:dbl)
                    n2634 = local read "Add up Stroke"() -> (w3210:dbl)
                    n2635 = call "FILE PATH CREATION.vi"("error in"=w3220, "FILE NAME :"=w3215) -> ("FILE OUT"=w3218:path)  [unwired: 8 in, 1 out]
                    n2636 = local read "STROKE Initialize"() -> (w3205:bool)
                    n2637 = Concatenate Strings(w3215, ".dgf" ("Substring")) -> (w3219:string)
                    n2638 = Subtract(x=w3212, y=w3210) -> (x-y=w3211:dbl)
                    n2639 = Absolute Value(x=w3211) -> (abs(x)=w3208:dbl)
                    n2640 = local read "FF 2"() -> (→"Frictional Force ( N )" →"Frictional Force ( N )":dbl)
                    n2641 = Build Path(base path=w3218, name or relative path=w3219) -> (appended path=w3214:path)
                    n2642 = flat-sequence {
                      tunnel: w3208 -> [w3274]
                      tunnel: [w3273] -> w3206
                      tunnel: w3205 -> [w3271]
                      tunnel: [w3276] -> w3207
                      tunnel: w3206 -> [w3276]
                      frame #0 {
                        n2643 = call <vilib>:"Mean PtByPt.vi"("x"=w3274, "sample length"="STROKE FILTER", "initialize"=w3271) -> ("mean"=w3273:dbl)  [unwired: 1 in, 1 out]
                      }
                      frame #1 {
                        "STROKE Initialize" <- FALSE ("STROKE Initialize")
                      }
                    }
                    n2644 = local read "COF 2"() -> (w3228:dbl)
                    "Coefficient of Friction" <- w3228
                    "COF 4" <- w3228
                    "Coefficient of Friction" <- w3228
                    n2645 = local read "TEMP"() -> (w3231:dbl)
                    "Temperature ( Deg C )" <- w3231
                    n2646 = local read "Humidity ( %RH )"() -> (w3230:dbl)
                    n2647 = local read "Frequency ( Hz )"() -> (w3237:dbl)
                    n2648 = local read "LVDT STROKE DISPLAY"() -> (w3209:dbl)